vi "FlexMag - 24-03-2023.vi"() -> ()   [LabVIEW 2018] (continued)
          }
          frame True {
            n14275 = stacked-sequence {
              frame #0 {
                n14276 = Two Button Dialog(message="Continue Chamber 3 Shut Down Process ?", 1:"No, Cancel" ("F button name (\"Cancel\")"), 2:"Yes, Continue" ("T button name (\"OK\")")) -> (T button?=→"ch3 sd continue":bool)
              }
              frame #1 {
                n14277 = Wait (ms)(milliseconds to wait=u32 100) -> ()  [unwired: 1 out]
              }
              frame #2 {
                n14278 = local read "ch3 sd continue"() -> (w19110:bool)
                n14279 = Wait (ms)(milliseconds to wait=u32 100) -> ()  [unwired: 1 out]
                n14280 = case shown="False" w19110 {
                  frame False {
                    w19111 = FALSE ("ch1 pumpdown alg")
                    n14281 = local write "ch3 shutdown alg"(w19111) -> ()
                    n14282 = local write "Shut Down CH3"(w19111) -> ()
                  }
                  frame True {
                    n14283 = local write "ch3 shutdown alg"(TRUE ("ch1 pumpdown alg")) -> ()
                  }
                }
              }
              frame #3 {
                n14284 = Wait (ms)(milliseconds to wait=u32 100) -> ()  [unwired: 1 out]
              }
              frame #4 {
                n14285 = local write "ch3 sd continue"(FALSE ("ch1 pd continue")) -> ()
              }
            }
          }
        }
        n14286 = case shown="True" w18994 {
          frame False {
          }
          frame True {
            n14287 = stacked-sequence {
              frame #0 {
                n14288 = Two Button Dialog(message="Cancel Chamber 3 Shut Down Process ?", 1:"No, Contunie" ("F button name (\"Cancel\")"), 2:"Yes, Cancel" ("T button name (\"OK\")")) -> (T button?=→"ch3 sd cancel":bool)
              }
              frame #1 {
                n14289 = Wait (ms)(milliseconds to wait=u32 100) -> ()  [unwired: 1 out]
              }
              frame #2 {
                n14290 = local read "ch3 sd cancel"() -> (w19099:bool)
                n14291 = Wait (ms)(milliseconds to wait=u32 100) -> ()  [unwired: 1 out]
                n14292 = case shown="True" w19099 {
                  frame False {
                    w19100 = TRUE ("ch1 pumpdown alg")
                    n14293 = local write "ch3 shutdown alg"(w19100) -> ()
                    n14294 = local write "Shut Down CH3"(w19100) -> ()
                  }
                  frame True {
                    w19101 = FALSE ("ch1 pumpdown alg")
                    n14295 = local write "ch3 shutdown alg"(w19101) -> ()
                    n14296 = local write "Shut Down CH3"(w19101) -> ()
                  }
                }
              }
              frame #3 {
                n14297 = Wait (ms)(milliseconds to wait=u32 100) -> ()  [unwired: 1 out]
              }
              frame #4 {
                n14298 = local write "ch3 sd cancel"(FALSE ("ch1 pd continue")) -> ()
              }
            }
          }
        }
        n14299 = local read "ch4 pumpdown alg"() -> (w19027:bool)
        n14300 = local read "ch4 pumpdown alg"() -> (w19037:bool)
        n14301 = local read "ch4 shutdown alg"() -> (w18983:bool)
        n14302 = local read "ch4 shutdown alg"() -> (w18984:bool)
        n14303 = feedback #320() -> (w19034:bool)  [unwired: 1 in]
        n14304 = feedback-in #320("Pump Down CH4") -> ()
        n14305 = feedback #321() -> (w18991:bool)  [unwired: 1 in]
        n14306 = feedback-in #321("Shut Down CH4") -> ()
        n14307 = Implies(1:w19034, 2:"Pump Down CH4") -> (0:w19031:bool)
        n14308 = Implies(1:w18991, 2:"Shut Down CH4") -> (0:w18988:bool)
        n14309 = Implies(1:"Pump Down CH4", 2:w19034) -> (0:w19029:bool)
        n14310 = Implies(1:"Shut Down CH4", 2:w18991) -> (0:w18986:bool)
        n14311 = Not(x=w19031) -> (.not. x?=w19032:bool)
        n14312 = Not(x=w18988) -> (.not. x?=w18989:bool)
        n14313 = Not(x=w19029) -> (.not. x?=w19033:bool)
        n14314 = Not(x=w19027) -> (.not. x?=w19030:bool)
        n14315 = Not(x=w18986) -> (.not. x?=w18990:bool)
        n14316 = Not(x=w18983) -> (.not. x?=w18987:bool)
        n14317 = Compound Arithmetic op=AND(w19033, w19037) -> (w19036:bool)
        n14318 = Compound Arithmetic op=AND(w19030, w19032) -> (w19035:bool)
        n14319 = Compound Arithmetic op=AND(w18990, w18984) -> (w18993:bool)
        n14320 = Compound Arithmetic op=AND(w18987, w18989) -> (w18992:bool)
        n14321 = case shown="True" w19035 {
          frame False {
          }
          frame True {
            n14322 = stacked-sequence {
              frame #0 {
                n14323 = Two Button Dialog(message="Continue Chamber 4 Pump Down Process ?", 1:"No, Cancel" ("F button name (\"Cancel\")"), 2:"Yes, Continue" ("T button name (\"OK\")")) -> (T button?=→"ch4 pd continue":bool)
              }
              frame #1 {
                n14324 = Wait (ms)(milliseconds to wait=u32 100) -> ()  [unwired: 1 out]
              }
              frame #2 {
                n14325 = local read "ch4 pd continue"() -> (w19176:bool)
                n14326 = Wait (ms)(milliseconds to wait=u32 100) -> ()  [unwired: 1 out]
                n14327 = case shown="False" w19176 {
                  frame False {
                    w19177 = FALSE ("ch1 pumpdown alg")
                    n14328 = local write "ch4 pumpdown alg"(w19177) -> ()
                    n14329 = local write "Pump Down CH4"(w19177) -> ()
                  }
                  frame True {
                    n14330 = local write "ch4 pumpdown alg"(TRUE ("ch1 pumpdown alg")) -> ()
                  }
                }
              }
              frame #3 {
                n14331 = Wait (ms)(milliseconds to wait=u32 100) -> ()  [unwired: 1 out]
              }
              frame #4 {
                n14332 = local write "ch4 pd continue"(FALSE ("ch1 pd continue")) -> ()
              }
            }
          }
        }
        n14333 = case shown="True" w19036 {
          frame False {
          }
          frame True {
            n14334 = stacked-sequence {
              frame #0 {
                n14335 = Two Button Dialog(message="Cancel Chamber 4 Pump Down Process ?", 1:"No, Contunie" ("F button name (\"Cancel\")"), 2:"Yes, Cancel" ("T button name (\"OK\")")) -> (T button?=→"ch4 pd cancel":bool)
              }
              frame #1 {
                n14336 = Wait (ms)(milliseconds to wait=u32 100) -> ()  [unwired: 1 out]
              }
              frame #2 {
                n14337 = local read "ch4 pd cancel"() -> (w19165:bool)
                n14338 = Wait (ms)(milliseconds to wait=u32 100) -> ()  [unwired: 1 out]
                n14339 = case shown="True" w19165 {
                  frame False {
                    w19166 = TRUE ("ch1 pumpdown alg")
                    n14340 = local write "ch4 pumpdown alg"(w19166) -> ()
                    n14341 = local write "Pump Down CH4"(w19166) -> ()
                  }
                  frame True {
                    w19167 = FALSE ("ch1 pumpdown alg")
                    n14342 = local write "ch4 pumpdown alg"(w19167) -> ()
                    n14343 = local write "Pump Down CH4"(w19167) -> ()
                  }
                }
              }
              frame #3 {
                n14344 = Wait (ms)(milliseconds to wait=u32 100) -> ()  [unwired: 1 out]
              }
              frame #4 {
                n14345 = local write "ch4 pd cancel"(FALSE ("ch1 pd continue")) -> ()
              }
            }
          }
        }
        n14346 = case shown="True" w18992 {
          frame False {
          }
          frame True {
            n14347 = stacked-sequence {
              frame #0 {
                n14348 = Two Button Dialog(message="Continue Chamber 4 Shut Down Process ?", 1:"No, Cancel" ("F button name (\"Cancel\")"), 2:"Yes, Continue" ("T button name (\"OK\")")) -> (T button?=→"ch4 sd continue":bool)
              }
              frame #1 {
                n14349 = Wait (ms)(milliseconds to wait=u32 100) -> ()  [unwired: 1 out]
              }
              frame #2 {
                n14350 = local read "ch4 sd continue"() -> (w19088:bool)
                n14351 = Wait (ms)(milliseconds to wait=u32 100) -> ()  [unwired: 1 out]
                n14352 = case shown="True" w19088 {
                  frame False {
                    w19089 = FALSE ("ch1 pumpdown alg")
                    n14353 = local write "ch4 shutdown alg"(w19089) -> ()
                    n14354 = local write "Shut Down CH4"(w19089) -> ()
                  }
                  frame True {
                    n14355 = local write "ch4 shutdown alg"(TRUE ("ch1 pumpdown alg")) -> ()
                  }
                }
              }
              frame #3 {
                n14356 = Wait (ms)(milliseconds to wait=u32 100) -> ()  [unwired: 1 out]
              }
              frame #4 {
                n14357 = local write "ch4 sd continue"(FALSE ("ch1 pd continue")) -> ()
              }
            }
          }
        }
        n14358 = case shown="True" w18993 {
          frame False {
          }
          frame True {
            n14359 = stacked-sequence {
              frame #0 {
                n14360 = Two Button Dialog(message="Cancel Chamber 4 Shut Down Process ?", 1:"No, Contunie" ("F button name (\"Cancel\")"), 2:"Yes, Cancel" ("T button name (\"OK\")")) -> (T button?=→"ch4 sd cancel":bool)
              }
              frame #1 {
                n14361 = Wait (ms)(milliseconds to wait=u32 100) -> ()  [unwired: 1 out]
              }
              frame #2 {
                n14362 = local read "ch4 sd cancel"() -> (w19077:bool)
                n14363 = Wait (ms)(milliseconds to wait=u32 100) -> ()  [unwired: 1 out]
                n14364 = case shown="False" w19077 {
                  frame False {
                    w19078 = TRUE ("ch1 pumpdown alg")
                    n14365 = local write "ch4 shutdown alg"(w19078) -> ()
                    n14366 = local write "Shut Down CH4"(w19078) -> ()
                  }
                  frame True {
                    w19079 = FALSE ("ch1 pumpdown alg")
                    n14367 = local write "ch4 shutdown alg"(w19079) -> ()
                    n14368 = local write "Shut Down CH4"(w19079) -> ()
                  }
                }
              }
              frame #3 {
                n14369 = Wait (ms)(milliseconds to wait=u32 100) -> ()  [unwired: 1 out]
              }
              frame #4 {
                n14370 = local write "ch4 sd cancel"(FALSE ("ch1 pd continue")) -> ()
              }
            }
          }
        }
      }
      frame True {
      }
    }
  }
  n14371 = disable-structure shown="Disabled" {
    frame Disabled {
      n14372 = stacked-sequence {
        frame #0 {
          n14373 = Get Date/Time String(date format (0)=enum16{"short", "long", "abbreviated"}."abbreviated", want seconds? (F)=TRUE) -> (date string=w19250:string)  [unwired: 1 in, 1 out]
          n14374 = Match Pattern(string=w19250, regular expression=", ") -> (after substring=w19255:string)  [unwired: 1 in, 3 out]
          n14375 = Path To String(path=path "E:/VK-1701 System Files/Pressure Text Files" ("start path")) -> (string=w19254:string)
          n14376 = Concatenate Strings(w19254, "\\" ("string"), w19255) -> (w19256:string)
          n14377 = String To Path(string=w19256) -> (path=w19257:path)
          n14378 = Open/Create/Replace File(file path (use dialog)=w19257, operation (0:open)=T16."open or create") -> ()  [unwired: 4 in, 3 out]
        }
        frame #1 {
          n14379 = while {
            stop <- FALSE stop-if-true
            n14380 = stacked-sequence {
              tunnel: [w19262 _] -> _
              frame #0 {
                n14381 = Get Date/Time String(date format (0)=enum16{"short", "long", "abbreviated"}."short", want seconds? (F)=TRUE) -> (date string=w19283:string, time string=w19286:string)  [unwired: 1 in]
                n14382 = local read "CH1 CH CC"() -> (w19360:string)
                n14383 = local read "CH1 CH PG"() -> (w19359:string)
                n14384 = local read "CH1 CH BG"() -> (w19363:string)
                n14385 = local read "CH1 PL PG"() -> (w19361:string)
                n14386 = Concatenate Strings(w19283, "\t", w19286, "\t") -> (w19279:string)
                n14387 = Concatenate Strings(w19279, "CH1 CH CC" ("text"), "\t", ":" ("text"), "\t", w19360, "\r\n") -> (w19278:string)
                n14388 = Concatenate Strings(w19279, "CH1 CH PG" ("text"), "\t", ":" ("text"), "\t", w19359, "\r\n") -> (w19277:string)
                n14389 = Concatenate Strings(w19279, "CH1 PL PG" ("text"), "\t", ":" ("text"), "\t", w19361, "\r\n") -> (w19276:string)
                n14390 = Concatenate Strings(w19279, "CH1 CH BG" ("text"), "\t", ":" ("text"), "\t", w19363, "\r\n") -> (w19275:string)
                n14391 = local read "CH1 CH CC"() -> (w19353:string)
                n14392 = local read "CH1 CH PG"() -> (w19354:string)
                n14393 = local read "CH1 CH BG"() -> (w19350:string)
                n14394 = local read "CH1 PL PG"() -> (w19352:string)
                n14395 = Concatenate Strings(w19279, "CH2 CH CC" ("text"), "\t", ":" ("text"), "\t", w19353, "\r\n") -> (w19274:string)
                n14396 = Concatenate Strings(w19279, "CH2 CH PG" ("text"), "\t", ":" ("text"), "\t", w19354, "\r\n") -> (w19273:string)
                n14397 = Concatenate Strings(w19279, "CH2 PL PG" ("text"), "\t", ":" ("text"), "\t", w19352, "\r\n") -> (w19272:string)
                n14398 = Concatenate Strings(w19279, "CH2 CH BG" ("text"), "\t", ":" ("text"), "\t", w19350, "\r\n") -> (w19271:string)
                n14399 = local read "CH1 CH CC"() -> (w19307:string)
                n14400 = local read "CH1 CH PG"() -> (w19308:string)
                n14401 = local read "CH1 CH BG"() -> (w19304:string)
                n14402 = local read "CH1 PL PG"() -> (w19306:string)
                n14403 = Concatenate Strings(w19279, "CH3 CH CC" ("text"), "\t", ":" ("text"), "\t", w19307, "\r\n") -> (w19270:string)
                n14404 = Concatenate Strings(w19279, "CH3 CH PG" ("text"), "\t", ":" ("text"), "\t", w19308, "\r\n") -> (w19269:string)
                n14405 = Concatenate Strings(w19279, "CH3 PL PG" ("text"), "\t", ":" ("text"), "\t", w19306, "\r\n") -> (w19268:string)  [unwired: 1 in]
                n14406 = Concatenate Strings(w19279, "CH3 CH BG" ("text"), "\t", ":" ("text"), "\t", w19304, "\r\n") -> (w19267:string)
                n14407 = local read "CH1 CH CC"() -> (w19314:string)
                n14408 = local read "CH1 CH PG"() -> (w19313:string)
                n14409 = local read "CH1 CH BG"() -> (w19317:string)
                n14410 = local read "CH1 PL PG"() -> (w19315:string)
                n14411 = Concatenate Strings(w19279, "CH4 CH CC" ("text"), "\t", ":" ("text"), "\t", w19314, "\r\n") -> (w19266:string)
                n14412 = Concatenate Strings(w19279, "CH4 CH PG" ("text"), "\t", ":" ("text"), "\t", w19313, "\r\n") -> (w19265:string)
                n14413 = Concatenate Strings(w19279, "CH4 PL PG" ("text"), "\t", ":" ("text"), "\t", w19315, "\r\n") -> (w19264:string)  [unwired: 1 in]
                n14414 = Concatenate Strings(w19279, "CH4 CH BG" ("text"), "\t", ":" ("text"), "\t", w19317, "\r\n") -> (w19263:string)
                n14415 = Concatenate Strings(w19278, w19277, w19276, w19275, w19274, w19273, w19272, w19271, w19270, w19269, w19268, w19267, w19266, w19265, w19264, w19263) -> (w19262:string)
              }
              frame #1 {
              }
            }
            n14416 = Wait Until Next ms Multiple(millisecond multiple=u32 1000) -> ()  [unwired: 1 out]
          }
        }
      }
    }
    frame Enabled {
    }
  }
  n14417 = while {
    stop <- FALSE stop-if-true
    n14418 = Wait Until Next ms Multiple(millisecond multiple=u32 300) -> ()  [unwired: 1 out]
    n14419 = case shown="True" "ch4 pumpdown alg" {
      frame False {
      }
      frame True {
        n14420 = local read "abort ch4"() -> (w19695:bool)
        n14421 = case shown="False" w19695 {
          frame False {
            n14422 = stacked-sequence {
              frame #0 {
                n14423 = stacked-sequence {
                  frame #0 {
                    n14424 = local write "ch4 pd clear"(TRUE ("ch1 pd clear")) -> ()
                    n14425 = Wait (ms)(milliseconds to wait=u32 100) -> ()  [unwired: 1 out]
                  }
                  frame #1 {
                    n14426 = local write "System Status"("CH4 PUMPDOWN PROCESS IN PROGRESS" ("System Status")) -> ()
                  }
                  frame #2 {
                    n14427 = local read "CH4_DS_DI"() -> (w19699:bool)
                    n14428 = case shown="True" w19699 {
                      frame False {
                      }
                      frame True {
                        n14429 = stacked-sequence {
                          frame #0 {
                            n14430 = local write "Buzzer DO"(TRUE ("Buzzer DO")) -> ()
                            n14431 = Wait (ms)(milliseconds to wait=u32 100) -> ()  [unwired: 1 out]
                          }
                          frame #1 {
                            n14432 = while {
                              i -> [w19704]
                              stop <- w19707 stop-if-true
                              n14433 = Greater?(x=w19704, y=900) -> (0:w19703:bool)
                              n14434 = case shown="True" w19703 {
                                frame False {
                                }
                                frame True {
                                n14435 = local write "Warning Message"("CH4 PumpDown process  is canceled !\nCH4 Door is open" ("Warning Message")) -> ()
                                n14436 = local write "ch4 pumpdown error"(TRUE ("ch1 pumpdown error")) -> ()
                                }
                              }
                              n14437 = local read "CH4_DS_DI"() -> (w19702:bool)
                              n14438 = case shown="True" w19702 {
                                tunnel: [FALSE TRUE] -> w19706
                                frame False {
                                n14439 = Wait Until Next ms Multiple(millisecond multiple=u32 200) -> ()  [unwired: 1 out]
                                }
                                frame True {
                                n14440 = local write "Buzzer DO"(FALSE ("Buzzer DO")) -> ()
                                }
                              }
                              n14441 = local read "ch4 pumpdown alg"() -> (w19708:bool)
                              n14442 = local read "abort ch4"() -> (w19710:bool)
                              n14443 = Not(x=w19708) -> (.not. x?=w19709:bool)
                              n14444 = Compound Arithmetic op=OR(w19706, w19710, w19709) -> (w19707:bool)
                            }
                          }
                        }
                      }
                    }
                  }
                  frame #3 {
                    n14445 = disable-structure shown="Disabled" {
                      frame Disabled {
                        n14446 = while {
                          i -> [w19719]
                          stop <- w19722 stop-if-true
                          n14447 = Greater?(x=w19719, y=900) -> (0:w19718:bool)
                          n14448 = case shown="True" w19718 {
                            frame False {
                            }
                            frame True {
                              n14449 = local write "Warning Message"("CH4 PumpDown process  is canceled !\nCH4 Water Switch couldn't be opened" ("Warning Message")) -> ()
                              n14450 = local write "ch4 pumpdown error"(TRUE ("ch1 pumpdown error")) -> ()
                            }
                          }
                          n14451 = local read "CH4_WFC_DI"() -> (w19717:bool)
                          n14452 = case shown="False" w19717 {
                            tunnel: [FALSE TRUE] -> w19721
                            frame False {
                              n14453 = Wait Until Next ms Multiple(millisecond multiple=u32 200) -> ()  [unwired: 1 out]
                              n14454 = local write "CH4_WFC_DO"(TRUE ("CH1_WFC_DO")) -> ()
                            }
                            frame True {
                            }
                          }
                          n14455 = local read "ch4 pumpdown alg"() -> (w19723:bool)
                          n14456 = local read "abort ch4"() -> (w19725:bool)
                          n14457 = Not(x=w19723) -> (.not. x?=w19724:bool)
                          n14458 = Compound Arithmetic op=OR(w19721, w19725, w19724) -> (w19722:bool)
                        }
                      }
                      frame Enabled {
                      }
                    }
                  }
                }
              }
              frame #1 {
                # "ATM switches close"
                n14459 = local read "ch4 pumpdown alg"() -> (w19732:bool)
                n14460 = case shown="True" w19732 {
                  frame False {
                  }
                  frame True {
                    n14461 = local read "abort ch4"() -> (w19733:bool)
                    n14462 = case shown="False" w19733 {
                      frame False {
                        w19735 = FALSE ("CH1_PL_ATM_DO")
                        n14463 = local write "CH4_PL_ATM_DO"(w19735) -> ()
                        n14464 = local write "CH4_CH_ATM_DO"(w19735) -> ()
                        n14465 = Wait (ms)(milliseconds to wait=u32 3000) -> ()  [unwired: 1 out]
                      }
                      frame True {
                      }
                    }
                  }
                }
              }
              frame #2 {
                n14466 = local read "ch4 pumpdown alg"() -> (w19736:bool)
                n14467 = case shown="True" w19736 {
                  frame False {
                  }
                  frame True {
                    n14468 = local read "abort ch4"() -> (w19737:bool)
                    n14469 = case shown="False" w19737 {
                      frame False {
                        n14470 = local write "ch4 atms close led"(TRUE ("CH1_PL_ATM_DO")) -> ()
                        n14471 = Wait (ms)(milliseconds to wait=u32 1000) -> ()  [unwired: 1 out]
                      }
                      frame True {
                      }
                    }
                  }
                }
              }
              frame #3 {
                # "ch vbv close"
                n14472 = local read "ch4 pumpdown alg"() -> (w19740:bool)
                n14473 = case shown="True" w19740 {
                  frame False {
                  }
                  frame True {
                    n14474 = local read "abort ch4"() -> (w19741:bool)
                    n14475 = case shown="False" w19741 {
                      frame False {
                        n14476 = while {
                          i -> [w19744]
                          stop <- w19747 stop-if-true
                          n14477 = Greater Or Equal?(x=w19744, y=100) -> (x >= y?=w19745:bool)
                          n14478 = case shown="True" w19745 {
                            frame False {
                            }
                            frame True {
                              n14479 = local write "Warning Message"("CH4 PumpDown process  is canceled !\nCH4 CH VBV couldn't be closed" ("Warning Message")) -> ()
                              n14480 = local write "ch4 pumpdown error"(TRUE ("ch1 pumpdown error")) -> ()
                            }
                          }
                          n14481 = local read "CH4_CH_VBV_DI"() -> (w19742:bool)
                          n14482 = local read "ch4 pumpdown alg"() -> (w19750:bool)
                          n14483 = case shown="True" w19742 {
                            tunnel: [TRUE FALSE] -> w19746
                            frame False {
                            }
                            frame True {
                              n14484 = local write "CH4_CH_VBV_DO"(FALSE ("CH1_CH_VBV_DO")) -> ()
                              n14485 = Wait Until Next ms Multiple(millisecond multiple=u32 200) -> ()  [unwired: 1 out]
                            }
                          }
                          n14486 = local read "abort ch4"() -> (w19748:bool)
                          n14487 = Not(x=w19750) -> (.not. x?=w19749:bool)
                          n14488 = Compound Arithmetic op=OR(w19746, w19748, w19749) -> (w19747:bool)
                        }
                      }
                      frame True {
                      }
                    }
                  }
                }
              }
              frame #4 {
                n14489 = local read "ch4 pumpdown alg"() -> (w19757:bool)
                n14490 = case shown="True" w19757 {
                  frame False {
                  }
                  frame True {
                    n14491 = local read "abort ch4"() -> (w19758:bool)
                    n14492 = case shown="False" w19758 {
                      frame False {
                        n14493 = local write "ch4 ch vbv close led"(TRUE ("ch1 ch vbv close")) -> ()
                        n14494 = Wait (ms)(milliseconds to wait=u32 1000) -> ()  [unwired: 1 out]
                      }
                      frame True {
                      }
                    }
                  }
                }
              }
              frame #5 {
                # "pl vbv close"
                n14495 = local read "ch4 pumpdown alg"() -> (w19761:bool)
                n14496 = case shown="True" w19761 {
                  frame False {
                  }
                  frame True {
                    n14497 = local read "abort ch4"() -> (w19762:bool)
                    n14498 = case shown="False" w19762 {
                      frame False {
                        n14499 = while {
                          i -> [w19765]
                          stop <- w19768 stop-if-true
                          n14500 = Greater Or Equal?(x=w19765, y=100) -> (x >= y?=w19766:bool)
                          n14501 = case shown="True" w19766 {
                            frame False {
                            }
                            frame True {
                              n14502 = local write "Warning Message"("CH4 PumpDown process  is canceled !\nCH4 PL VBV couldn't be closed" ("Warning Message")) -> ()
                              n14503 = local write "ch4 pumpdown error"(TRUE ("ch1 pumpdown error")) -> ()
                            }
                          }
                          n14504 = local read "CH4_PL_VBV_DI"() -> (w19763:bool)
                          n14505 = local read "ch4 pumpdown alg"() -> (w19771:bool)
                          n14506 = case shown="True" w19763 {
                            tunnel: [TRUE FALSE] -> w19767
                            frame False {
                            }
                            frame True {
                              n14507 = Wait Until Next ms Multiple(millisecond multiple=u32 200) -> ()  [unwired: 1 out]
                              n14508 = local write "CH4_PL_VBV_DO"(FALSE ("CH1_CH_VBV_DO")) -> ()
                            }
                          }
                          n14509 = local read "abort ch4"() -> (w19769:bool)
                          n14510 = Not(x=w19771) -> (.not. x?=w19770:bool)
                          n14511 = Compound Arithmetic op=OR(w19767, w19769, w19770) -> (w19768:bool)
                        }
                      }
                      frame True {
                      }
                    }
                  }
                }
              }
              frame #6 {
                n14512 = local read "ch4 pumpdown alg"() -> (w19778:bool)
                n14513 = case shown="True" w19778 {
                  frame False {
                  }
                  frame True {
                    n14514 = local read "abort ch4"() -> (w19779:bool)
                    n14515 = case shown="False" w19779 {
                      frame False {
                        n14516 = local write "ch4 pl vbv close led"(TRUE ("ch1 ch vbv close")) -> ()
                        n14517 = Wait (ms)(milliseconds to wait=u32 1000) -> ()  [unwired: 1 out]
                      }
                      frame True {
                      }
                    }
                  }
                }
              }
              frame #7 {
                n14518 = local read "ch4 pumpdown alg"() -> (w19782:bool)
                n14519 = case shown="True" w19782 {
                  frame False {
                  }
                  frame True {
                    n14520 = local read "abort ch4"() -> (w19783:bool)
                    n14521 = case shown="False" w19783 {
                      frame False {
                        n14522 = local read "ch3 ch pg torr"() -> (w19788:dbl)
                        n14523 = local read "CH4_CH_ATM_DI"() -> (w19787:bool)
                        n14524 = Less?(x=w19788, y=0.5) -> (x < y?=w19786:bool)
                        n14525 = And(x=w19787, y=w19786) -> (x .and. y?=w19784:bool)
                        n14526 = case shown="False" w19784 {
                          frame False {
                            # "ch trns bp right close"
                            n14527 = while {
                              i -> [w19791]
                              stop <- w19794 stop-if-true
                              n14528 = Greater Or Equal?(x=w19791, y=100) -> (x >= y?=w19792:bool)
                              n14529 = case shown="True" w19792 {
                                frame False {
                                }
                                frame True {
                                n14530 = local write "Warning Message"("CH4 PumpDown process  is canceled !\nCH4 TRNS BP Right couldn't be closed" ("Warning Message")) -> ()
                                n14531 = local write "ch4 pumpdown error"(TRUE ("ch1 pumpdown error")) -> ()
                                }
                              }
                              n14532 = local read "CH4_Trns_BP_Right_DI"() -> (w19789:bool)
                              n14533 = local read "ch4 pumpdown alg"() -> (w19797:bool)
                              n14534 = case shown="True" w19789 {
                                tunnel: [TRUE FALSE] -> w19793
                                frame False {
                                }
                                frame True {
                                n14535 = local write "CH4_Trns_BP_Right_DO"(FALSE ("CH1_CH_VBV_DO")) -> ()
                                n14536 = Wait Until Next ms Multiple(millisecond multiple=u32 200) -> ()  [unwired: 1 out]
                                }
                              }
                              n14537 = local read "abort ch4"() -> (w19795:bool)
                              n14538 = Not(x=w19797) -> (.not. x?=w19796:bool)
                              n14539 = Compound Arithmetic op=OR(w19793, w19795, w19796) -> (w19794:bool)
                            }
                          }
                          frame True {
                            # "ch trns bp right open"
                            n14540 = while {
                              i -> [w19806]
                              stop <- w19809 stop-if-true
                              n14541 = Greater Or Equal?(x=w19806, y=100) -> (x >= y?=w19807:bool)
                              n14542 = case shown="True" w19807 {
                                frame False {
                                }
                                frame True {
                                n14543 = local write "Warning Message"("CH4 PumpDown process  is canceled !\nCH4 TRNS BP Right couldn't be open" ("Warning Message")) -> ()
                                n14544 = local write "ch4 pumpdown error"(TRUE ("ch1 pumpdown error")) -> ()
                                }
                              }
                              n14545 = local read "CH4_Trns_BP_Right_DI"() -> (w19804:bool)
                              n14546 = local read "ch4 pumpdown alg"() -> (w19812:bool)
                              n14547 = case shown="False" w19804 {
                                tunnel: [FALSE TRUE] -> w19808
                                frame False {
                                n14548 = local write "CH4_Trns_BP_Right_DO"(TRUE ("CH1_CH_VBV_DO")) -> ()
                                n14549 = Wait Until Next ms Multiple(millisecond multiple=u32 200) -> ()  [unwired: 1 out]
                                }
                                frame True {
                                }
                              }
                              n14550 = local read "abort ch4"() -> (w19810:bool)
                              n14551 = Not(x=w19812) -> (.not. x?=w19811:bool)
                              n14552 = Compound Arithmetic op=OR(w19808, w19810, w19811) -> (w19809:bool)
                            }
                          }
                        }
                      }
                      frame True {
                      }
                    }
                  }
                }
              }
              frame #8 {
                n14553 = local read "ch4 pumpdown alg"() -> (w19819:bool)
                n14554 = case shown="True" w19819 {
                  frame False {
                  }
                  frame True {
                    n14555 = local read "abort ch4"() -> (w19820:bool)
                    n14556 = case shown="False" w19820 {
                      frame False {
                        n14557 = local read "CH4_Trns_BP_Right_DI"() -> (w19821:bool)
                        n14558 = case shown="False" w19821 {
                          frame False {
                            n14559 = local write "ch4 trns bp right close led"(TRUE ("ch1 ch vbv close")) -> ()
                            n14560 = Wait (ms)(milliseconds to wait=u32 1000) -> ()  [unwired: 1 out]
                          }
                          frame True {
                          }
                        }
                      }
                      frame True {
                      }
                    }
                  }
                }
              }
              frame #9 {
                # "ch trns gv 3-4 close"
                n14561 = local read "ch4 pumpdown alg"() -> (w19824:bool)
                n14562 = case shown="True" w19824 {
                  frame False {
                  }
                  frame True {
                    n14563 = local read "abort ch4"() -> (w19825:bool)
                    n14564 = case shown="False" w19825 {
                      frame False {
                        n14565 = while {
                          i -> [w19828]
                          stop <- w19831 stop-if-true
                          n14566 = Greater Or Equal?(x=w19828, y=100) -> (x >= y?=w19829:bool)
                          n14567 = case shown="True" w19829 {
                            frame False {
                            }
                            frame True {
                              n14568 = local write "Warning Message"("CH3 PumpDown process  is canceled !\nCH3-CH4 TRNS GV couldn't be closed" ("Warning Message")) -> ()
                              n14569 = local write "ch4 pumpdown error"(TRUE ("ch1 pumpdown error")) -> ()
                            }
                          }
                          n14570 = local read "CH3_Trns_Gv_Close_DI"() -> (w19826:bool)
                          n14571 = case shown="False" w19826 {
                            tunnel: [FALSE TRUE] -> w19830
                            frame False {
                              n14572 = local write "CH3_Trns_GV_Open_DO"(FALSE ("CH3_Trns_GV_Open_DO")) -> ()
                              n14573 = local write "CH3_Trns_GV_Close_DO"(TRUE ("CH1_CH_VBV_DO")) -> ()
                              n14574 = Wait Until Next ms Multiple(millisecond multiple=u32 200) -> ()  [unwired: 1 out]
                            }
                            frame True {
                            }
                          }
                          n14575 = local read "ch4 pumpdown alg"() -> (w19834:bool)
                          n14576 = local read "abort ch4"() -> (w19832:bool)
                          n14577 = Not(x=w19834) -> (.not. x?=w19833:bool)
                          n14578 = Compound Arithmetic op=OR(w19830, w19832, w19833) -> (w19831:bool)
                        }
                      }
                      frame True {
                      }
                    }
                  }
                }
              }
              frame #10 {
                n14579 = local read "ch4 pumpdown alg"() -> (w19842:bool)
                n14580 = case shown="True" w19842 {
                  frame False {
                  }
                  frame True {
                    n14581 = local read "abort ch4"() -> (w19843:bool)
                    n14582 = case shown="False" w19843 {
                      frame False {
                        n14583 = local write "ch4-ch3 trns gv close led"(TRUE ("ch1 ch vbv close")) -> ()
                        n14584 = Wait (ms)(milliseconds to wait=u32 1000) -> ()  [unwired: 1 out]
                      }
                      frame True {
                      }
                    }
                  }
                }
              }
              frame #11 {
                # "tp bv open\npc gv open"
                n14585 = local read "ch4 pumpdown alg"() -> (w19846:bool)
                n14586 = case shown="True" w19846 {
                  frame False {
                  }
                  frame True {
                    n14587 = local read "abort ch4"() -> (w19847:bool)
                    n14588 = case shown="False" w19847 {
                      frame False {
                        n14589 = local read "CH4_CH_ATM_DI"() -> (w19849:bool)
                        n14590 = local read "CH4_PL_ATM_DI"() -> (w19850:bool)
                        n14591 = And(x=w19849, y=w19850) -> (x .and. y?=w19848:bool)
                        n14592 = case shown="True" w19848 {
                          frame False {
                          }
                          frame True {
                            n14593 = stacked-sequence {
                              frame #0 {
                                # "tp bv open\npc gv open"
                              }
                              frame #1 {
                                n14594 = while {
                                i -> [w19853]
                                stop <- w19856 stop-if-true
                                n14595 = Greater Or Equal?(x=w19853, y=100) -> (x >= y?=w19854:bool)
                                n14596 = case shown="True" w19854 {
                                frame False {
                                }
                                frame True {
                                n14597 = local write "Warning Message"("CH4 PumpDown process  is canceled !\nCH4 TP BV couldn't be opened" ("Warning Message")) -> ()
                                n14598 = local write "ch4 pumpdown error"(TRUE ("ch1 pumpdown error")) -> ()
                                }
                                }
                                n14599 = local read "CH4_TP_BV_DI"() -> (w19851:bool)
                                n14600 = local read "ch4 pumpdown alg"() -> (w19859:bool)
                                n14601 = case shown="False" w19851 {
                                tunnel: [FALSE TRUE] -> w19855
                                frame False {
                                n14602 = Wait Until Next ms Multiple(millisecond multiple=u32 200) -> ()  [unwired: 1 out]
                                n14603 = local write "CH4_TP_BV_DO"(TRUE ("CH1_CH_VBV_DO")) -> ()
                                }
                                frame True {
                                }
                                }
                                n14604 = local read "abort ch4"() -> (w19857:bool)
                                n14605 = Not(x=w19859) -> (.not. x?=w19858:bool)
                                n14606 = Compound Arithmetic op=OR(w19855, w19857, w19858) -> (w19856:bool)
                                }
                              }
                              frame #2 {
                                n14607 = local read "ch4 pumpdown alg"() -> (w19866:bool)
                                n14608 = case shown="True" w19866 {
                                frame False {
                                }
                                frame True {
                                n14609 = local write "ch4 tp bv open led"(TRUE ("ch1 tp bv open led")) -> ()
                                n14610 = Wait (ms)(milliseconds to wait=u32 1000) -> ()  [unwired: 1 out]
                                }
                                }
                              }
                              frame #3 {
                                n14611 = stacked-sequence {
                                frame #0 {
                                n14612 = local read "ch4 pumpdown alg"() -> (w19869:bool)
                                n14613 = case shown="True" w19869 {
                                frame False {
                                }
                                frame True {
                                n14614 = flat-sequence {
                                frame #0 {
                                n14615 = local write "pcgv4 auto open"(TRUE ("pcgv1 auto open")) -> ()
                                }
                                frame #1 {
                                n14616 = Wait (ms)(milliseconds to wait=u32 2000) -> ()  [unwired: 1 out]
                                }
                                frame #2 {
                                n14617 = local write "pcgv4 auto open"(TRUE ("pcgv1 auto open")) -> ()
                                }
                                }
                                }
                                }
                                }
                                frame #1 {
                                n14618 = while {
                                i -> [w19879]
                                stop <- w19875 stop-if-true
                                n14619 = Greater Or Equal?(x=w19879, y=200) -> (x >= y?=w19881:bool)
                                n14620 = case shown="True" w19881 {
                                frame False {
                                }
                                frame True {
                                n14621 = local write "ch4 pumpdown error"(TRUE ("ch1 pumpdown error")) -> ()
                                n14622 = local write "Warning Message"("CH4 PumpDown process  is canceled !\nCH4 PC GV couldn't be opened" ("Warning Message")) -> ()
                                }
                                }
                                n14623 = local read "ch4 pumpdown alg"() -> (w19878:bool)
                                n14624 = local read "ch4_pcgv_gui"() -> (w19874:bool)
                                n14625 = local read "abort ch4"() -> (w19876:bool)
                                n14626 = Wait Until Next ms Multiple(millisecond multiple=u32 200) -> ()  [unwired: 1 out]
                                n14627 = Not(x=w19878) -> (.not. x?=w19877:bool)
                                n14628 = Compound Arithmetic op=OR(w19874, w19876, w19877) -> (w19875:bool)
                                }
                                }
                                }
                              }
                              frame #4 {
                                n14629 = local read "ch4 pumpdown alg"() -> (w19884:bool)
                                n14630 = case shown="True" w19884 {
                                frame False {
                                }
                                frame True {
                                n14631 = local write "ch4 pc gv open led"(TRUE ("ch1 tp bv open led")) -> ()
                                n14632 = Wait (ms)(milliseconds to wait=u32 1000) -> ()  [unwired: 1 out]
                                }
                                }
                              }
                            }
                          }
                        }
                      }
                      frame True {
                      }
                    }
                  }
                }
              }
              frame #12 {
                n14633 = stacked-sequence {
                  frame #0 {
                    n14634 = local read "ch4 pumpdown alg"() -> (w19887:bool)
                    n14635 = case shown="True" w19887 {
                      frame False {
                      }
                      frame True {
                        n14636 = local read "abort ch4"() -> (w19888:bool)
                        n14637 = case shown="False" w19888 {
                          frame False {
                            n14638 = local write "CH4_PL_ATM_DO"(TRUE ("CH1_PL_ATM_DO")) -> ()
                            n14639 = Wait (ms)(milliseconds to wait=u32 2000) -> ()  [unwired: 1 out]
                          }
                          frame True {
                          }
                        }
                      }
                    }
                  }
                  frame #1 {
                    n14640 = local read "ch4 pumpdown alg"() -> (w19891:bool)
                    n14641 = case shown="True" w19891 {
                      frame False {
                      }
                      frame True {
                        n14642 = local read "abort ch4"() -> (w19892:bool)
                        n14643 = case shown="False" w19892 {
                          frame False {
                            n14644 = local write "CH4_CH_ATM_DO"(TRUE ("CH1_CH_ATM_DO")) -> ()
                            n14645 = Wait (ms)(milliseconds to wait=u32 2000) -> ()  [unwired: 1 out]
                          }
                          frame True {
                          }
                        }
                      }
                    }
                  }
                }
              }
              frame #13 {
                # "mp start"
                n14646 = local read "ch4 pumpdown alg"() -> (w19895:bool)
                n14647 = case shown="True" w19895 {
                  frame False {
                  }
                  frame True {
                    n14648 = local read "abort ch4"() -> (w19896:bool)
                    n14649 = case shown="False" w19896 {
                      frame False {
                        n14650 = while {
                          i -> [w19901]
                          stop <- w19905 stop-if-true
                          n14651 = Greater?(x=w19901, y=100) -> (0:w19897:bool)
                          n14652 = case shown="True" w19897 {
                            frame False {
                            }
                            frame True {
                              n14653 = local write "Warning Message"("CH4 PumpDown process  is canceled !\nCH4 MP couldn't be started" ("Warning Message")) -> ()
                              n14654 = local write "ch4 pumpdown error"(TRUE ("ch1 pumpdown error")) -> ()
                            }
                          }
                          n14655 = local read "CH4_MP_DI"() -> (w19899:bool)
                          n14656 = case shown="False" w19899 {
                            tunnel: [FALSE TRUE] -> w19898
                            frame False {
                              n14657 = Wait Until Next ms Multiple(millisecond multiple=u32 200) -> ()  [unwired: 1 out]
                              n14658 = local write "CH4_MP_DO"(TRUE ("CH1_MP_DO")) -> ()
                            }
                            frame True {
                            }
                          }
                          n14659 = local read "ch4 pumpdown alg"() -> (w19904:bool)
                          n14660 = local read "abort ch4"() -> (w19902:bool)
                          n14661 = Not(x=w19904) -> (.not. x?=w19903:bool)
                          n14662 = Compound Arithmetic op=OR(w19898, w19902, w19903) -> (w19905:bool)
                        }
                      }
                      frame True {
                      }
                    }
                  }
                }
              }
              frame #14 {
                n14663 = local read "ch4 pumpdown alg"() -> (w19912:bool)
                n14664 = case shown="True" w19912 {
                  frame False {
                  }
                  frame True {
                    n14665 = local read "abort ch4"() -> (w19913:bool)
                    n14666 = case shown="False" w19913 {
                      frame False {
                        n14667 = local write "ch4 mp start led"(TRUE ("ch1 ch vbv close")) -> ()
                        n14668 = Wait (ms)(milliseconds to wait=u32 1000) -> ()  [unwired: 1 out]
                      }
                      frame True {
                      }
                    }
                  }
                }
              }
              frame #15 {
                # "pl pg check"
                n14669 = local read "ch4 pumpdown alg"() -> (w19916:bool)
                n14670 = case shown="True" w19916 {
                  frame False {
                  }
                  frame True {
                    n14671 = local read "abort ch4"() -> (w19917:bool)
                    n14672 = case shown="False" w19917 {
                      frame False {
                        n14673 = while {
                          i -> [w19924]
                          stop <- w19928 stop-if-true
                          # "30 min"
                          n14674 = Greater?(x=w19924, y=9000) -> (0:w19921:bool)
                          n14675 = case shown="True" w19921 {
                            frame False {
                            }
                            frame True {
                              n14676 = local write "Warning Message"("CH4 PumpDown process  is canceled !\nCH4 PL Pressure couldn't reach under 0.05 Torr" ("Warning Message")) -> ()
                              n14677 = local write "ch4 pumpdown error"(TRUE ("ch1 pumpdown error")) -> ()
                            }
                          }
                          n14678 = local read "ch4 pl pg torr"() -> (w19920:dbl)
                          n14679 = Less?(x=w19920, y=0.7) -> (x < y?=w19918:bool)
                          n14680 = case shown="False" w19918 {
                            tunnel: [FALSE TRUE] -> w19922
                            frame False {
                              n14681 = Wait Until Next ms Multiple(millisecond multiple=u32 200) -> ()  [unwired: 1 out]
                            }
                            frame True {
                            }
                          }
                          n14682 = local read "ch4 pumpdown alg"() -> (w19927:bool)
                          n14683 = local read "abort ch4"() -> (w19925:bool)
                          n14684 = Not(x=w19927) -> (.not. x?=w19926:bool)
                          n14685 = Compound Arithmetic op=OR(w19922, w19925, w19926) -> (w19928:bool)
                        }
                      }
                      frame True {
                      }
                    }
                  }
                }
              }
              frame #16 {
                n14686 = local read "ch4 pumpdown alg"() -> (w19934:bool)
                n14687 = case shown="True" w19934 {
                  frame False {
                  }
                  frame True {
                    n14688 = local read "abort ch4"() -> (w19935:bool)
                    n14689 = case shown="False" w19935 {
                      frame False {
                        n14690 = local write "ch4 pl press under 0.05 T led"(TRUE ("ch1 ch vbv close")) -> ()
                        n14691 = Wait (ms)(milliseconds to wait=u32 1000) -> ()  [unwired: 1 out]
                      }
                      frame True {
                      }
                    }
                  }
                }
              }
              frame #17 {
                # "tp bv open"
                n14692 = local read "ch4 pumpdown alg"() -> (w19938:bool)
                n14693 = case shown="True" w19938 {
                  frame False {
                  }
                  frame True {
                    n14694 = local read "abort ch4"() -> (w19939:bool)
                    n14695 = case shown="False" w19939 {
                      frame False {
                        n14696 = while {
                          i -> [w19944]
                          stop <- w19948 stop-if-true
                          n14697 = Greater?(x=w19944, y=100) -> (0:w19940:bool)
                          n14698 = case shown="True" w19940 {
                            frame False {
                            }
                            frame True {
                              n14699 = local write "Warning Message"("CH4 PumpDown process  is canceled !\nCH4 TP BV couldn't be opened" ("Warning Message")) -> ()
                              n14700 = local write "ch4 pumpdown error"(TRUE ("ch1 pumpdown error")) -> ()
                            }
                          }
                          n14701 = local read "CH4_TP_BV_DI"() -> (w19942:bool)
                          n14702 = case shown="False" w19942 {
                            tunnel: [FALSE TRUE] -> w19941
                            frame False {
                              n14703 = Wait Until Next ms Multiple(millisecond multiple=u32 200) -> ()  [unwired: 1 out]
                              n14704 = local write "CH4_TP_BV_DO"(TRUE ("CH1_MP_DO")) -> ()
                            }
                            frame True {
                            }
                          }
                          n14705 = local read "ch4 pumpdown alg"() -> (w19947:bool)
                          n14706 = local read "abort ch4"() -> (w19945:bool)
                          n14707 = Not(x=w19947) -> (.not. x?=w19946:bool)
                          n14708 = Compound Arithmetic op=OR(w19941, w19945, w19946) -> (w19948:bool)
                        }
                      }
                      frame True {
                      }
                    }
                  }
                }
              }
              frame #18 {
                n14709 = local read "ch4 pumpdown alg"() -> (w19955:bool)
                n14710 = case shown="True" w19955 {
                  frame False {
                  }
                  frame True {
                    n14711 = local read "abort ch4"() -> (w19956:bool)
                    n14712 = case shown="False" w19956 {
                      frame False {
                        n14713 = local write "ch4 tp bv open led"(TRUE ("ch1 ch vbv close")) -> ()
                        n14714 = Wait (ms)(milliseconds to wait=u32 1000) -> ()  [unwired: 1 out]
                      }
                      frame True {
                      }
                    }
                  }
                }
              }
              frame #19 {
                # "pc gv open"
                n14715 = local read "ch4 pumpdown alg"() -> (w19959:bool)
                n14716 = case shown="True" w19959 {
                  frame False {
                  }
                  frame True {
                    n14717 = local read "abort ch4"() -> (w19960:bool)
                    n14718 = case shown="False" w19960 {
                      frame False {
                        n14719 = stacked-sequence {
                          frame #0 {
                            n14720 = local read "ch4 pumpdown alg"() -> (w19961:bool)
                            n14721 = case shown="True" w19961 {
                              frame False {
                              }
                              frame True {
                                n14722 = flat-sequence {
                                frame #0 {
                                n14723 = local write "pcgv4 auto open"(TRUE ("pcgv1 auto open")) -> ()
                                }
                                frame #1 {
                                n14724 = Wait (ms)(milliseconds to wait=u32 2000) -> ()  [unwired: 1 out]
                                }
                                frame #2 {